vi "Velociprobe_Nanopositioner_Control_RT 2.vi"() -> ()   [LabVIEW 2015] (continued)
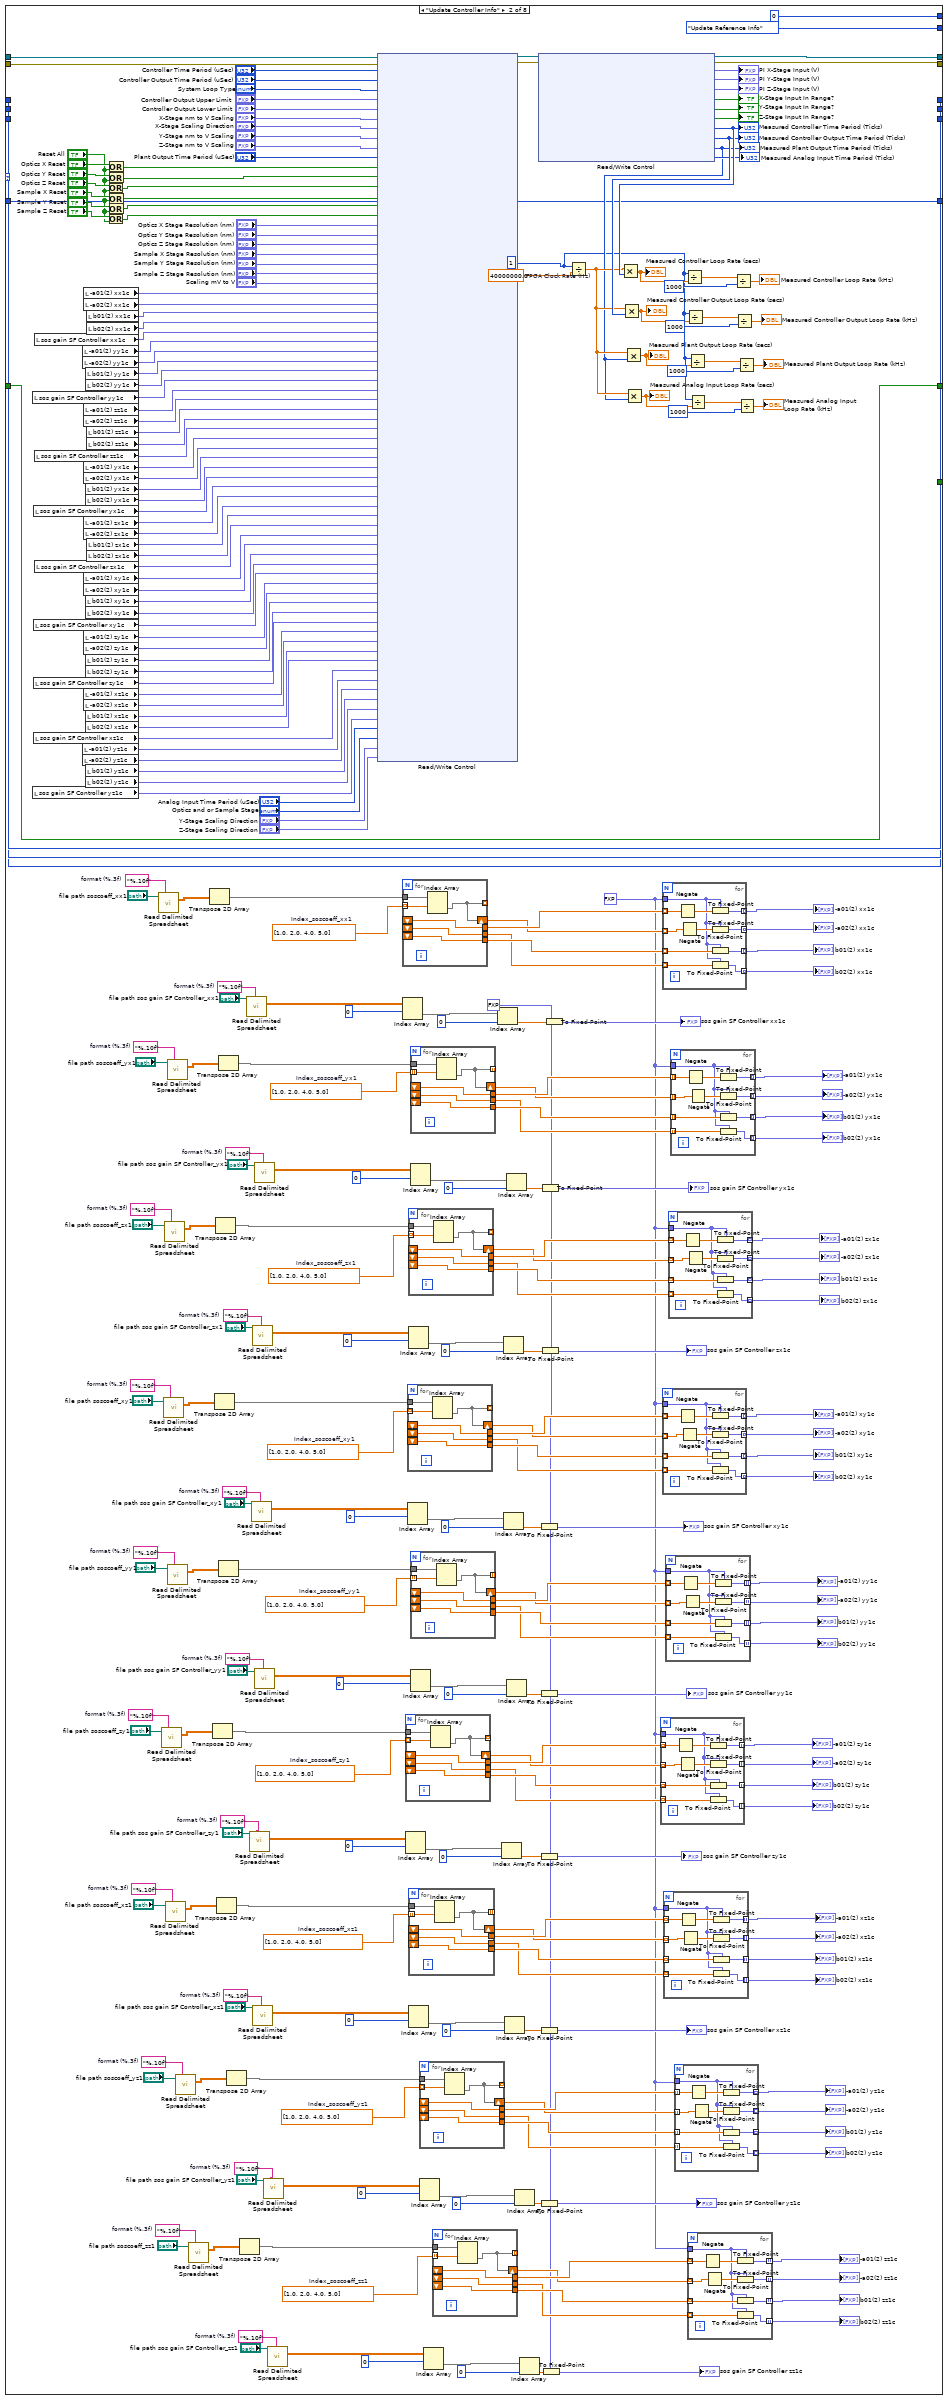
[diagram p2: hidden frame]
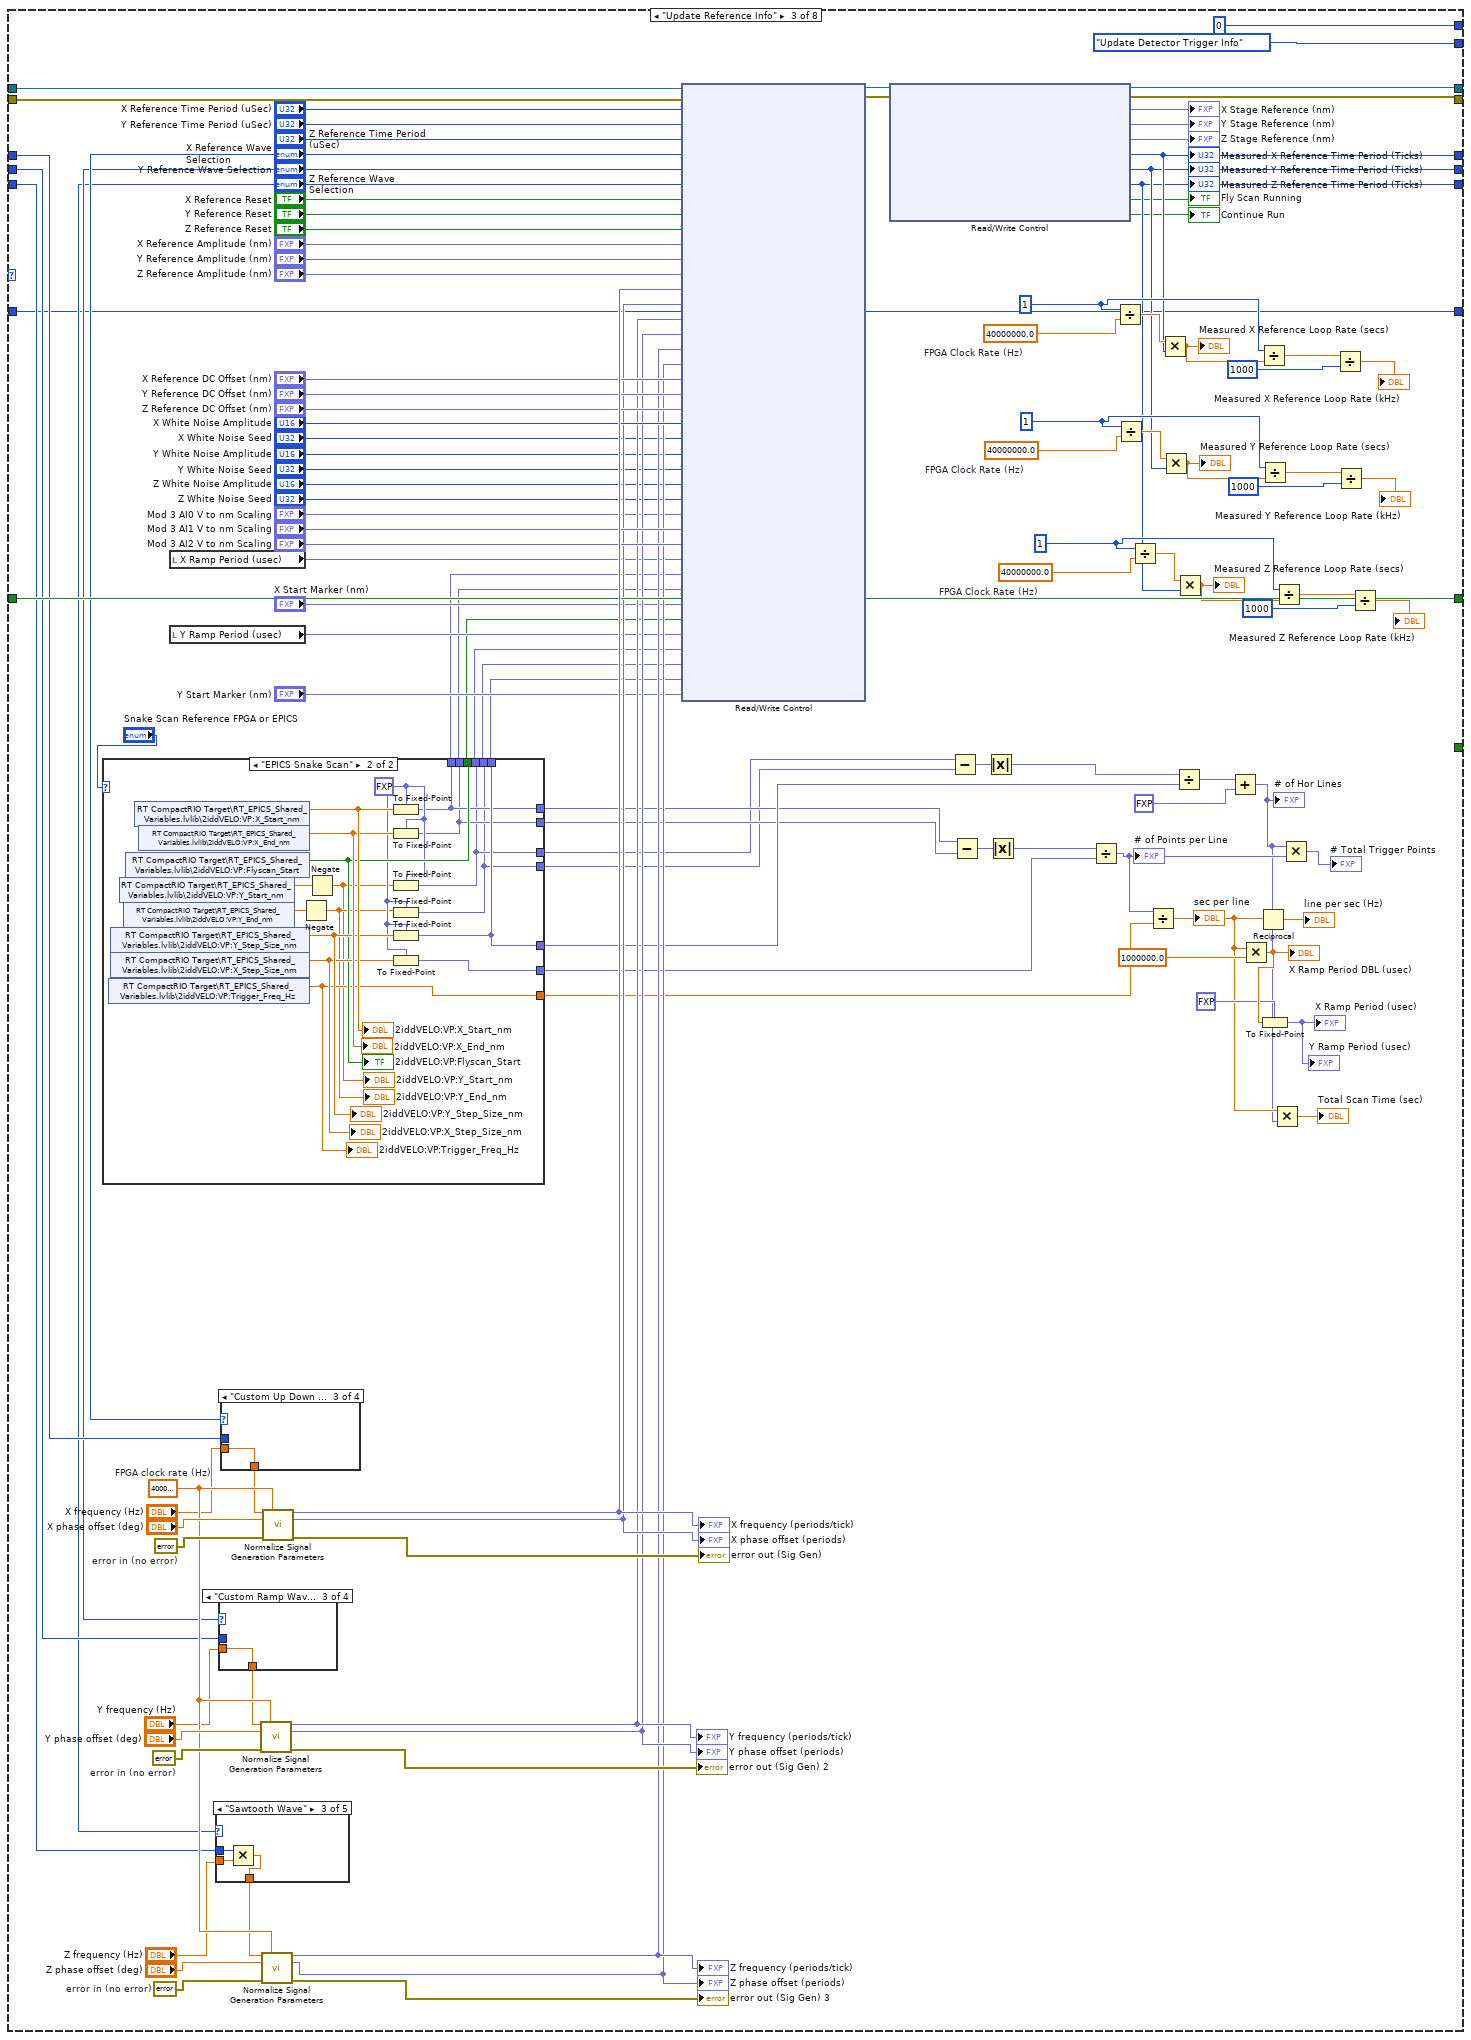
[diagram p3: hidden frame]
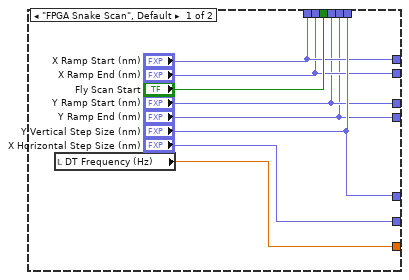
[diagram p4: hidden frame]
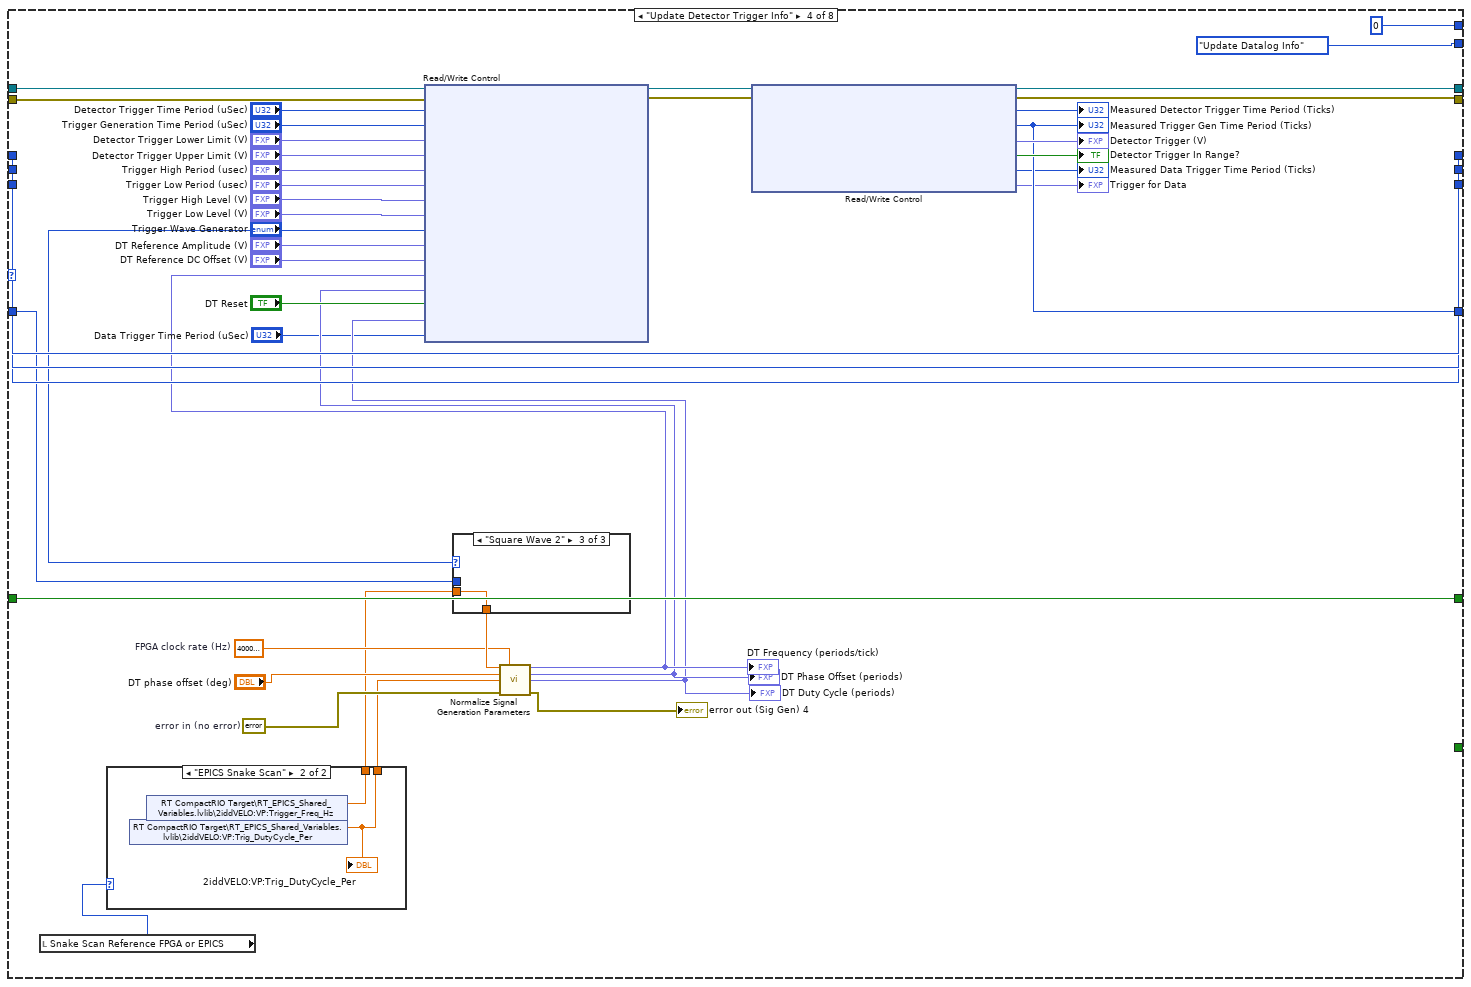
[diagram p15: hidden frame]
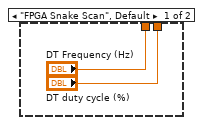
[diagram p16: hidden frame]
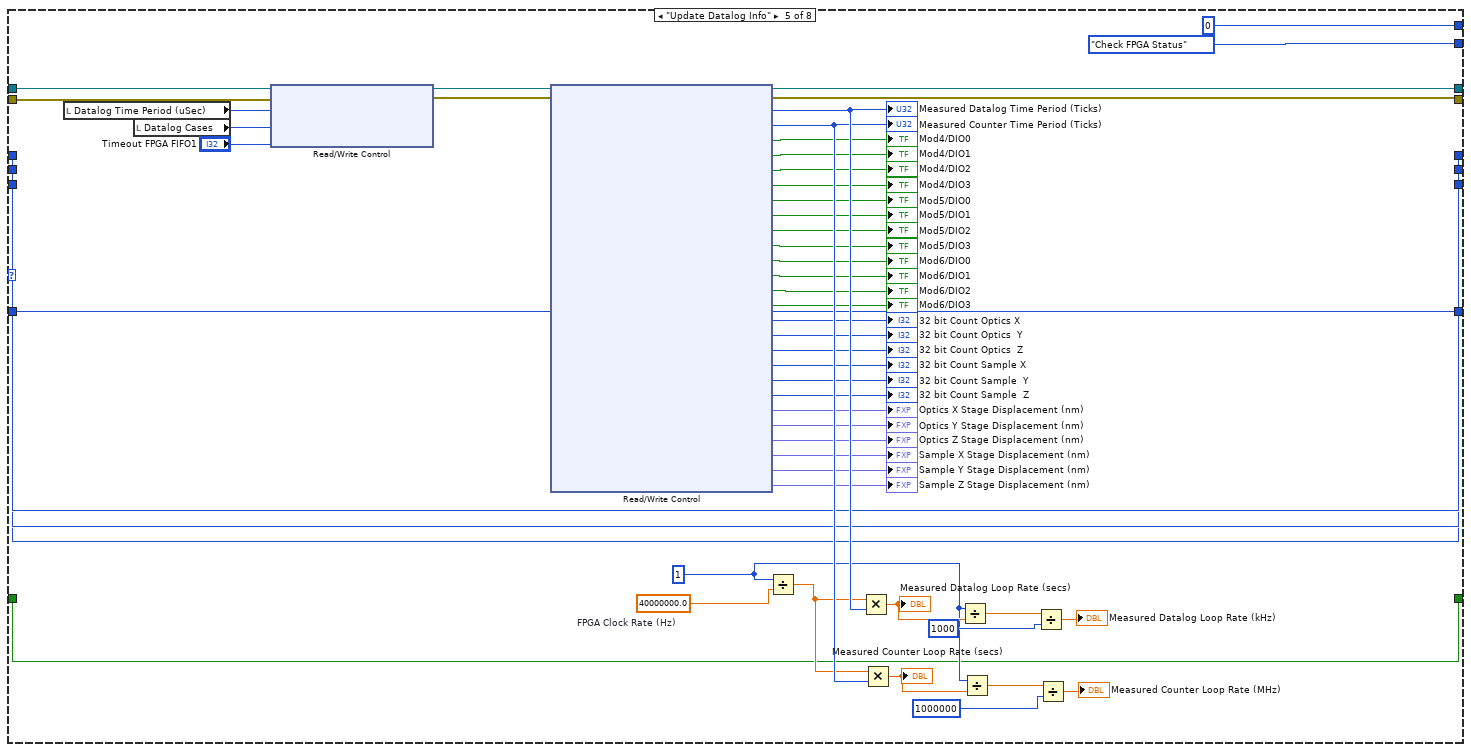
[diagram p19: hidden frame]
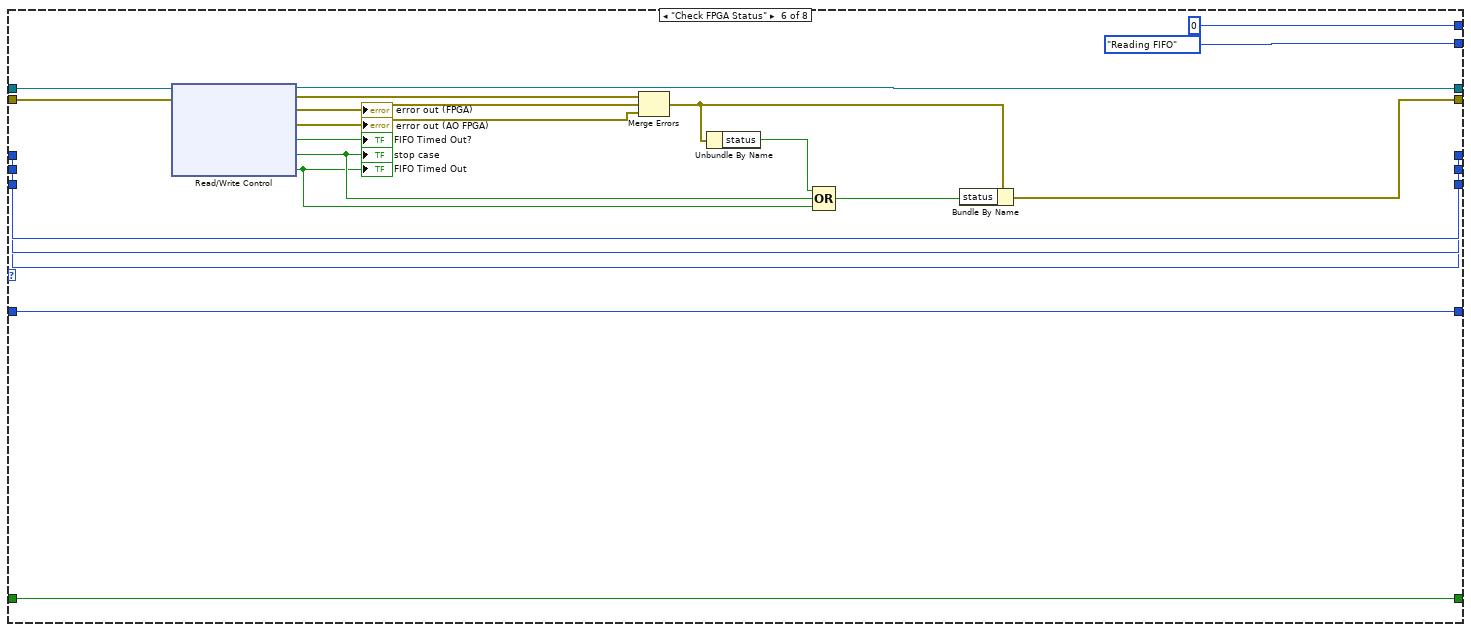
[diagram p20: hidden frame]
        n244 = xnode "Read/Write Control"("FPGA VI Reference In"=w537, "error in"=w536) -> ("FPGA VI Reference Out"=w534:refnum<k20>, "error out"=w535:errorcluster, "X Stage Reference (nm)"=→"X Stage Reference (nm)":fxp<+/-,58,25>, "Y Stage Reference (nm)"=→"Y Stage Reference (nm)":fxp<+/-,58,25>, "Z Stage Reference (nm)"=→"Z Stage Reference (nm)":fxp<+/-,58,25>, "Measured X Reference Time Period (Ticks)"=w583:u32, "Measured Y Reference Time Period (Ticks)"=w579:u32, "Measured Z Reference Time Period (Ticks)"=w578:u32, "Fly Scan Running"=→"Fly Scan Running":bool, "Continue Run"=→"Continue Run":bool)
        "Measured X Reference Time Period (Ticks)" <- w583
        "Measured Y Reference Time Period (Ticks)" <- w579
        "Measured Z Reference Time Period (Ticks)" <- w578
        n245 = Subtract(x=w530, y=w529) -> (x-y=w566:fxp<+/-,17,17>)
        n246 = Subtract(x=w532, y=w531) -> (x-y=w564:fxp<+/-,17,17>)
        n247 = Absolute Value(x=w566) -> (abs(x)=w557:fxp<+,16,16>)
        n248 = Absolute Value(x=w564) -> (abs(x)=w563:fxp<+,16,16>)
        n249 = Divide(x=w563, y=w541) -> (x/y=w561:fxp<+/-,33,17>)
        "# of Points per Line" <- w561
        n250 = Divide(x=w629, y=w635) -> (x/y=w630:dbl)
        n251 = Divide(x=w607, y=w613) -> (x/y=w608:dbl)
        n252 = Divide(x=w600, y=w606) -> (x/y=w601:dbl)
        n253 = Divide(x=w561, y=w540) -> (x/y=w553:dbl)
        "sec per line" <- w553
        n254 = Multiply(x=w630, y=w583) -> (x*y=w634:dbl)
        "Measured X Reference Loop Rate (secs)" <- w634
        n255 = Multiply(x=w608, y=w579) -> (x*y=w612:dbl)
        "Measured Y Reference Loop Rate (secs)" <- w612
        n256 = Divide(x=w557, y=w533) -> (x/y=w558:fxp<+/-,33,17>)
        n257 = Multiply(x=w601, y=w578) -> (x*y=w605:dbl)
        "Measured Z Reference Loop Rate (secs)" <- w605
        n258 = Add(x=w558, y=fxp<+,16,16> 1.0) -> (x+y=w552:fxp<+/-,34,18>)
        "# of Hor Lines" <- w552
        n259 = Multiply(x=w553, y=1000000.0) -> (x*y=w556:dbl)
        "X Ramp Period DBL (usec)" <- w556
        n260 = Reciprocal(x=w553) -> (1/x=→"line per sec (Hz)":dbl)
        n261 = Divide(x=w629, y=w634) -> (x/y=w633:dbl)
        n262 = Divide(x=w607, y=w612) -> (x/y=w611:dbl)
        n263 = To Fixed-Point(fixed-point type=fxp<+,24,24> 0.0, number=w556) -> (fixed-point=→"X Ramp Period (usec)" →"Y Ramp Period (usec)":fxp<+,24,24>)
        n264 = Multiply(x=w553, y=w552) -> (x*y=→"Total Scan Time (sec)":dbl)
        n265 = Divide(x=w600, y=w605) -> (x/y=w604:dbl)
        n266 = Multiply(x=w552, y=w561) -> (x*y=→"# Total Trigger Points":fxp<+/-,64,34>)
        n267 = Divide(x=w633, y=1000) -> (x/y=→"Measured X Reference Loop Rate (kHz)":dbl)
        n268 = Divide(x=w611, y=1000) -> (x/y=→"Measured Y Reference Loop Rate (kHz)":dbl)
        n269 = Divide(x=w604, y=1000) -> (x/y=→"Measured Z Reference Loop Rate (kHz)":dbl)
      }
      frame "Update Detector Trigger Info" {
        w709 = 40000000.0  # FPGA clock rate (Hz)
        w711 = errorcluster {"status"=FALSE, "code"=0, "source"=""}  # error in (no error)
        n270 = local read "Snake Scan Reference FPGA or EPICS"() -> (w702:enum16{"FPGA Snake Scan", "EPICS Snake Scan"})
        n271 = case shown="\"EPICS Snake Scan\"" w702 {
          tunnel: ["DT Frequency (Hz)" w737] -> w701
          tunnel: ["DT duty cycle (%)" w736] -> w700
          frame "FPGA Snake Scan", Default {
          }
          frame "EPICS Snake Scan" {
            n272 = shared-variable "RT CompactRIO Target\\RT_EPICS_Shared_Variables.lvlib\\2iddVELO:VP:Trig_DutyCycle_Per"() -> (w736:dbl)  [unwired: 1 in, 1 out]
            "2iddVELO:VP:Trig_DutyCycle_Per" <- w736
            n273 = shared-variable "RT CompactRIO Target\\RT_EPICS_Shared_Variables.lvlib\\2iddVELO:VP:Trigger_Freq_Hz"() -> (w737:dbl)  [unwired: 1 in, 1 out]
          }
        }
        n274 = case shown="\"Square Wave 2\"" "Trigger Wave Generator" {
          tunnel: w701 -> [w738 w739 w740]
          tunnel: [w738 w739 w740] -> w710
          tunnel: w703 -> [_ _ _]
          frame "Custom Square Wave ", Default {
          }
          frame "Square Wave 1" {
          }
          frame "Square Wave 2" {
          }
        }
        n275 = call <vilib>:"Normalize Signal Generation Parameters.vi"("frequency (Hz)"=w710, "FPGA clock rate (Hz)"=w709, "phase offset (deg)"="DT phase offset (deg)", "duty cycle (%)"=w700, "error in (no error)"=w711) -> ("frequency (periods/tick)"=w707:fxp<+,32,0>, "phase offset (periods)"=w706:fxp<+,32,0>, "duty cycle (periods)"=w705:fxp<+,32,0>, "error out"=→"error out (Sig Gen) 4":errorcluster)  [unwired: 5 in, 2 out]
        "DT Frequency (periods/tick)" <- w707
        "DT Phase Offset (periods)" <- w706
        "DT Duty Cycle (periods)" <- w705
        n276 = xnode "Read/Write Control"("FPGA VI Reference In"=w699, "error in"=w698, "Detector Trigger Time Period (uSec)"="Detector Trigger Time Period (uSec)", "Trigger Generation Time Period (uSec)"="Trigger Generation Time Period (uSec)", "Detector Trigger Lower Limit (V)"="Detector Trigger Lower Limit (V)", "Detector Trigger Upper Limit (V)"="Detector Trigger Upper Limit (V)", "Trigger High Period (usec)"="Trigger High Period (usec)", "Trigger Low Period (usec)"="Trigger Low Period (usec)", "Trigger High Level (V)"="Trigger High Level (V)", "Trigger Low Level (V)"="Trigger Low Level (V)", "Trigger Wave Generator"="Trigger Wave Generator", "DT Reference Amplitude (V)"="DT Reference Amplitude (V)", "DT Reference DC Offset (V)"="DT Reference DC Offset (V)", "DT Frequency (periods/tick)"=w707, "DT Phase Offset (periods)"=w706, "DT Reset"="DT Reset", "DT Duty Cycle (periods)"=w705, "Data Trigger Time Period (uSec)"="Data Trigger Time Period (uSec)") -> ("FPGA VI Reference Out"=w697:refnum<k20>, "error out"=w696:errorcluster)
        n277 = xnode "Read/Write Control"("FPGA VI Reference In"=w697, "error in"=w696) -> ("FPGA VI Reference Out"=w695:refnum<k20>, "error out"=w694:errorcluster, "Measured Detector Trigger Time Period (Ticks)"=→"Measured Detector Trigger Time Period (Ticks)":u32, "Measured Trigger Gen Time Period (Ticks)"=w704:u32, "Detector Trigger (V)"=→"Detector Trigger (V)":fxp<+/-,20,5>, "Detector Trigger In Range?"=→"Detector Trigger In Range?":bool, "Measured Data Trigger Time Period (Ticks)"=→"Measured Data Trigger Time Period (Ticks)":u32, "Trigger for Data"=→"Trigger for Data":fxp<+/-,58,25>)
        "Measured Trigger Gen Time Period (Ticks)" <- w704
      }
      frame "Update Datalog Info" {
        w785 = 40000000.0  # FPGA Clock Rate (Hz)
        w774 = 1
        n278 = local read "Datalog Time Period (uSec)"() -> (w772:u32)
        n279 = local read "Datalog Cases"() -> (w771:T7)
        n280 = xnode "Read/Write Control"("FPGA VI Reference In"=w746, "error in"=w745, "Datalog Time Period (uSec)"=w772, "Datalog Cases"=w771, "Timeout FPGA FIFO1"="Timeout FPGA FIFO1") -> ("FPGA VI Reference Out"=w744:refnum<k20>, "error out"=w743:errorcluster)
        n281 = xnode "Read/Write Control"("FPGA VI Reference In"=w744, "error in"=w743) -> ("FPGA VI Reference Out"=w741:refnum<k20>, "error out"=w742:errorcluster, "Measured Datalog Time Period (Ticks)"=w784:u32, "Measured Counter Time Period (Ticks)"=w782:u32, "Mod4/DIO0"=→"Mod4/DIO0":bool, "Mod4/DIO1"=→"Mod4/DIO1":bool, "Mod4/DIO2"=→"Mod4/DIO2":bool, "Mod4/DIO3"=→"Mod4/DIO3":bool, "Mod5/DIO0"=→"Mod5/DIO0":bool, "Mod5/DIO1"=→"Mod5/DIO1":bool, "Mod5/DIO2"=→"Mod5/DIO2":bool, "Mod5/DIO3"=→"Mod5/DIO3":bool, "Mod6/DIO0"=→"Mod6/DIO0":bool, "Mod6/DIO1"=→"Mod6/DIO1":bool, "Mod6/DIO2"=→"Mod6/DIO2":bool, "Mod6/DIO3"=→"Mod6/DIO3":bool, "32 bit Count Optics X"=→"32 bit Count Optics X":i32, "32 bit Count Optics  Y"=→"32 bit Count Optics  Y":i32, "32 bit Count Optics  Z"=→"32 bit Count Optics  Z":i32, "32 bit Count Sample X"=→"32 bit Count Sample X":i32, "32 bit Count Sample  Y"=→"32 bit Count Sample  Y":i32, "32 bit Count Sample  Z"=→"32 bit Count Sample  Z":i32, "Optics X Stage Displacement (nm)"=→"Optics X Stage Displacement (nm)":fxp<+/-,58,25>, "Optics Y Stage Displacement (nm)"=→"Optics Y Stage Displacement (nm)":fxp<+/-,58,25>, "Optics Z Stage Displacement (nm)"=→"Optics Z Stage Displacement (nm)":fxp<+/-,58,25>, "Sample X Stage Displacement (nm)"=→"Sample X Stage Displacement (nm)":fxp<+/-,58,25>, "Sample Y Stage Displacement (nm)"=→"Sample Y Stage Displacement (nm)":fxp<+/-,58,25>, "Sample Z Stage Displacement (nm)"=→"Sample Z Stage Displacement (nm)":fxp<+/-,58,25>)
        "Measured Datalog Time Period (Ticks)" <- w784
        "Measured Counter Time Period (Ticks)" <- w782
        n282 = Divide(x=w774, y=w785) -> (x/y=w781:dbl)
        n283 = Multiply(x=w781, y=w784) -> (x*y=w792:dbl)
        "Measured Datalog Loop Rate (secs)" <- w792
        n284 = Multiply(x=w781, y=w782) -> (x*y=w788:dbl)
        "Measured Counter Loop Rate (secs)" <- w788
        n285 = Divide(x=w774, y=w792) -> (x/y=w791:dbl)
        n286 = Divide(x=w774, y=w788) -> (x/y=w787:dbl)
        n287 = Divide(x=w791, y=1000) -> (x/y=→"Measured Datalog Loop Rate (kHz)":dbl)
        n288 = Divide(x=w787, y=1000000) -> (x/y=→"Measured Counter Loop Rate (MHz)":dbl)
      }
      frame "Check FPGA Status" {
        n289 = xnode "Read/Write Control"("FPGA VI Reference In"=w798, "error in"=w797) -> ("FPGA VI Reference Out"=w796:refnum<k20>, "error out"=w795:errorcluster, "error out (FPGA)"=w811:errorcluster, "error out (AO FPGA)"=w810:errorcluster, "FIFO Timed Out?"=→"FIFO Timed Out?":bool, "stop case"=w805:bool, "FIFO Timed Out"=w804:bool)
        "error out (FPGA)" <- w811
        "error out (AO FPGA)" <- w810
        "stop case" <- w805
        "FIFO Timed Out" <- w804
        n290 = Merge Errors "Merge Errors"(w795, w811, w810) -> (w806:errorcluster)
        n291 = Unbundle By Name "Unbundle By Name"(w806) -> ("status"=w809:bool)
        n292 = Compound Arithmetic op=OR(w809, w805, w804) -> (w807:bool)
        n293 = Bundle By Name "Bundle By Name"(cluster=w806, "status"=w807) -> (w794:errorcluster)
      }
      frame "Reading FIFO" {
        w865 = 0.0  # t0
        n294 = local read "Snake Scan Reference FPGA or EPICS"() -> (w818:enum16{"FPGA Snake Scan", "EPICS Snake Scan"})
        n295 = local read "Datalog Time Period (uSec)"() -> (w863:u32)
        n296 = xnode "Read/Write Control"("FPGA VI Reference In"=w826, "error in"=w825) -> ("FPGA VI Reference Out"=w824:refnum<k20>, "error out"=w823:errorcluster, "Number of Data Strings"=→"Number of Data Strings":i32)
        n297 = Multiply(x=1e-06, y=w863) -> (x*y=w855:dbl)
        "Datalog Time Period (sec)" <- w855
        n298 = Divide(x=1.0, y=w855) -> (x/y=w859:dbl)
        "Datalog Rate (Hz)" <- w859
        n299 = case shown="\"EPICS Snake Scan\"" w818 {
          tunnel: ["Write Data" w870] -> w817
          frame "FPGA Snake Scan", Default {
          }
          frame "EPICS Snake Scan" {
            n300 = shared-variable "RT CompactRIO Target\\RT_EPICS_Shared_Variables.lvlib\\2iddVELO:VP:Write_Data"() -> (w870:bool)  [unwired: 1 in, 1 out]
            "2iddVELO:VP:Write_Data" <- w870
          }
        }
        n301 = Multiply(x="FIFO Time Period", y=w859) -> (x*y=w857:dbl)
        n302 = Multiply(x=5 ("Number of Data Strings 2"), y=w857) -> (x*y=w856:dbl)
        n303 = To Unsigned Long Integer(number=w856) -> (unsigned 32bit integer=w852:u32)
        "Number of Elements" <- w852
        n304 = xnode "Invoke Method"("FPGA VI Reference In"=w824, "error in"=w823, "Number of Elements"=w852, "Timeout (ms)"="Timeout (ms)") -> ("FPGA VI Reference Out"=w822:refnum<k20>, "error out"=w821:errorcluster, "Data"=w853:fxp<+/-,58,25>[], "Elements Remaining"=→"Elements Remaining" →"Elements Remaining Waveform Chart" →"Elements Remaining Waveform Chart 3":u32)
        "Data" <- w853
        n305 = Greater?(x=w817, y=w851) -> (0:w848:bool)
        n306 = case shown="True" w848 {
          tunnel: w825 -> [w883 w886]
          tunnel: [w883 w887] -> w846
          frame False {
          }
          frame True {
            n307 = call "Data_Write.vi"("Command List"=Data_Write_Control."Initialize", "name"="name", "error initialize"=w886) -> ("error out"=w887:errorcluster)  [unwired: 6 in]
          }
        }
        n308 = Decimate 1D Array "Decimate 1D Array"(w853) -> (w840:fxp<+/-,58,25>[], w831:fxp<+/-,58,25>[], w830:fxp<+/-,58,25>[], w829:fxp<+/-,58,25>[], w827:fxp<+/-,58,25>[])
        n309 = Build Array "Build Array"(w840, w831, w830, w829, w827) -> (w866:fxp<+/-,58,25>[][])
        n310 = To Double Precision Float(number=w866) -> (double precision float=w861:dbl[][])
        n311 = Transpose 2D Array(2D array=w861) -> (transposed array=w844:dbl[][])
        n312 = case shown="True" w817 {
          tunnel: w846 -> [w875 w881]
          tunnel: [w875 w882] -> w845
          tunnel: w844 -> [_ w876]
          frame False {
          }
          frame True {
            w879 = "%8f"  # format string
            w878 = ","  # delimiter (Tab)
            n313 = Array To Spreadsheet String(delimiter (Tab)=w878, array=w876, 3:w879) -> (spreadsheet string=w877:string)
            n314 = call "Data_Write.vi"("Command List"=Data_Write_Control."Write", "Data"=w877, "error initialize"=w881) -> ("error out"=w882:errorcluster)  [unwired: 6 in]
          }
        }
        n315 = Bundle("t0"=w865, w855, w861) -> (→"Waveform Graph 2":cluster{"t0":dbl, dbl, dbl[][]})  [unwired: 1 in]
        n316 = call "Convert to Dynamic Data"("Array"=w840) -> ("Dynamic Data Type"=w838:dynamicdata)  [unwired: 3 in]
        n317 = call "Convert to Dynamic Data2"("Array"=w831) -> ("Dynamic Data Type"=w832:dynamicdata)  [unwired: 3 in]
        n318 = call "Convert to Dynamic Data3"("Array"=w830) -> ("Dynamic Data Type"=w834:dynamicdata)  [unwired: 3 in]
        n319 = call "Convert to Dynamic Data4"("Array"=w829) -> ("Dynamic Data Type"=w833:dynamicdata)  [unwired: 3 in]
        n320 = call "Convert from Dynamic Data"("Dynamic Data Type"=w838) -> ("Array"=w839:dbl[])  [unwired: 3 in]
        n321 = call "Convert from Dynamic Data2"("Dynamic Data Type"=w832) -> ("Array"=w837:dbl[])  [unwired: 3 in]
        n322 = call "Convert from Dynamic Data3"("Dynamic Data Type"=w834) -> ("Array"=w836:dbl[])  [unwired: 3 in]
        n323 = call "Convert from Dynamic Data4"("Dynamic Data Type"=w833) -> ("Array"=w835:dbl[])  [unwired: 3 in]
        n324 = Less?(x=w817, y=w851) -> (x < y?=w847:bool)
        n325 = Bundle("Array"=w839, "Array"=w837) -> (→"XY Graph":cluster{"Array":dbl[], "Array":dbl[]})  [unwired: 1 in]
        n326 = Bundle("Array"=w836, "Array"=w835) -> (→"XY Graph 2":cluster{"Array":dbl[], "Array":dbl[]})  [unwired: 1 in]
        n327 = case shown="True" w847 {
          tunnel: w845 -> [w871 w873]
          tunnel: [w871 w874] -> w854
          frame False {
          }
          frame True {
            n328 = call "Data_Write.vi"("Command List"=Data_Write_Control."Close", "error initialize"=w873) -> ("error out"=w874:errorcluster)  [unwired: 7 in]
          }
        }
        n329 = Merge Errors "Merge Errors"(w821, w854) -> (w820:errorcluster)
      }
      frame "Exit" {
        w900 = TRUE ("Stop")
        n330 = xnode "Invoke Method"("FPGA VI Reference In"=w894, "error in"=w893) -> ("FPGA VI Reference Out"=w892:refnum<k20>, "error out"=w891:errorcluster)
        n331 = xnode "Read/Write Control"("FPGA VI Reference In"=w892, "error in"=w891, "stop case"=TRUE) -> ("FPGA VI Reference Out"=w890:refnum<k20>, "error out"=w889:errorcluster)
        n332 = local write "Stop"(w900) -> ()
        n333 = xnode "Close FPGA VI Reference"("FPGA VI Reference In"=w890, "error in"=w889) -> ("error out"=w888:errorcluster)
      }
    }
    n334 = call "State Control.vi"("Error Input"=w14, "Input States"=w25, "Stop"="Stop") -> ("Output State"=w24:T8)  [unwired: 8 in]
    n335 = node-c288(w31) -> ()  [unwired: 1 out]
  }
  n336 = node-c288(w7) -> (→"Error (RT)":errorcluster, →"Iteration Duration RT Timed-Loop":i64)
  n337 = call <vilib>:"Simple Error Handler.vi"("error in (no error)"=w1) -> ("message"=→"message":string)  [unwired: 4 in, 4 out]
